vi "inject contour on intensity plot.vi"(5 "graph para":T1={"x offset"=-10.0, "y offset"=0.0, "x scale"=0.1, "y scale"=0.002}, 7 "Threshold":dbl, 11 "IV Intensity":dbl[][](array[numeric])=array201x1000[201000 elements]) -> (1 "Y":dbl[](array[numeric]), 2 "X":dbl[](array[numeric]), 3 "IV Intensity output":dbl[][](graph))   [LabVIEW 2024]
uses:
  graph para.ctl
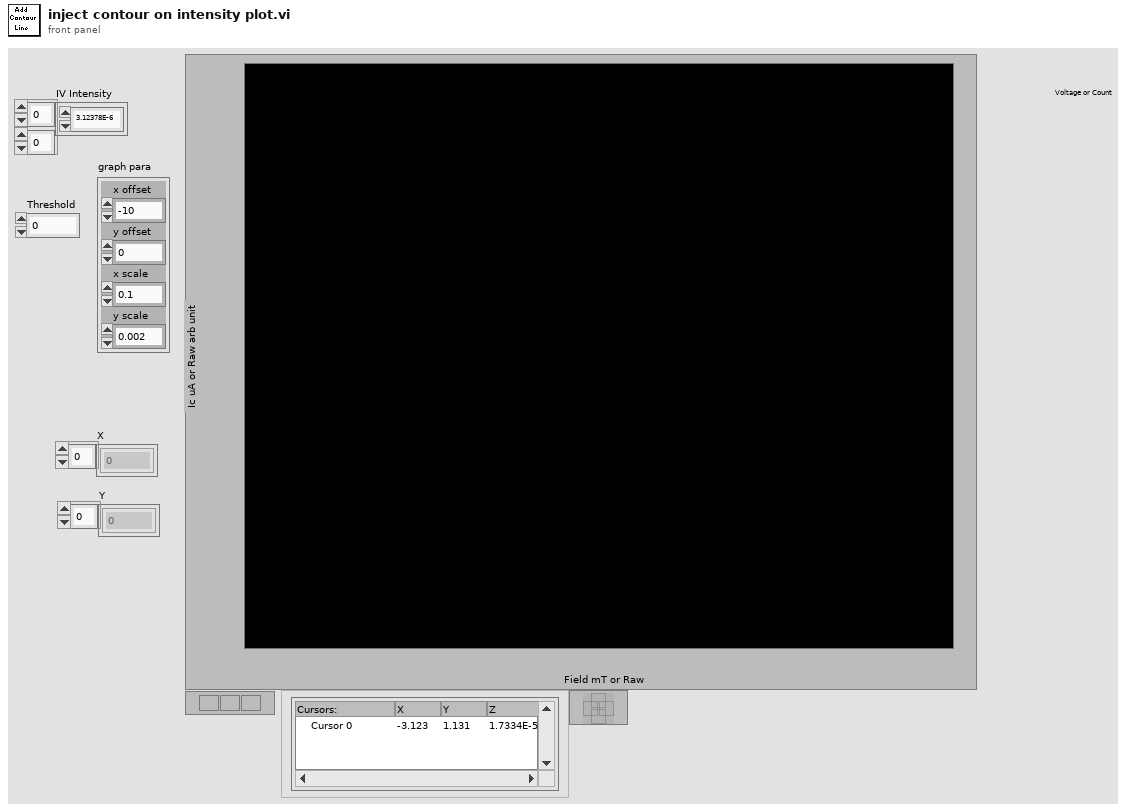
[diagram p1: front panel]
types:
  T1 = typedef "graph para.ctl" = cluster{"x offset":dbl, "y offset":dbl, "x scale":dbl, "y scale":dbl}
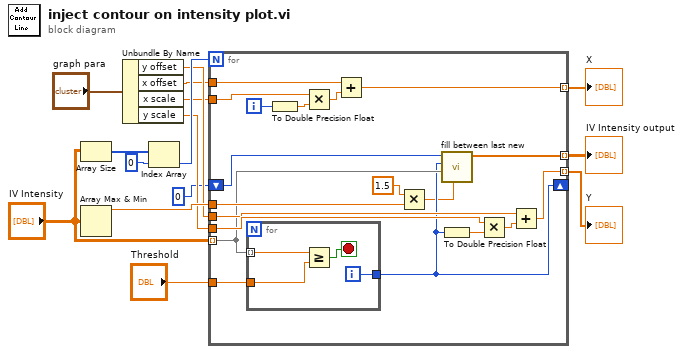
[diagram p0: block diagram]
diagram:
  n1 = Array Size(array="IV Intensity") -> (size(s)=w15:i32[])
  n2 = Array Max & Min(array="IV Intensity") -> (max value=w11:dbl)  [unwired: 3 out]
  n3 = Unbundle By Name("graph para") -> ("y offset"=w8:dbl, "x offset"=w7:dbl, "x scale"=w6:dbl, "y scale"=w5:dbl)
  n4 = Index Array(array=w15, index=0) -> (element=w13:i32)
  n5 = for {
    N: w13 -> [_]
    tunnel: w6 -> [w33]
    tunnel: w7 -> [w30]
    tunnel: w8 -> [w22]
    tunnel: w5 -> [w23]
    tunnel: "IV Intensity" -> [w20] mode=indexing
    tunnel: w11 -> [w29]
    tunnel: [w19] -> w10 mode=indexing
    tunnel: "Threshold" -> [w27]
    tunnel: [w26] -> w3 mode=indexing
    tunnel: [w21] -> w2 mode=indexing
    shift-right: [w17] -> _
    shift-left: 0 -> [w18]
    i -> [w34]
    n6 = for {
      tunnel: w20 -> [w38] mode=indexing
      tunnel: w27 -> [w37]
      tunnel: [w35] -> w17
      i -> [w35]
      stop <- w36 stop-if-true
      n7 = Greater Or Equal?(x=w38, y=w37) -> (x >= y?=w36:bool)
    }
    n8 = To Double Precision Float(number=w34) -> (double precision float=w32:dbl)
    n9 = Multiply(x=w33, y=w32) -> (x*y=w31:dbl)
    n10 = Add(x=w30, y=w31) -> (x+y=w26:dbl)
    n11 = Multiply(x=1.5, y=w29) -> (x*y=w16:dbl)
    n12 = call "fill between last new.vi"("value"=w16, "array in"=w20, "New"=w17, "Last"=w18) -> ("array out"=w19:dbl[])  [unwired: 7 in]
    n13 = To Double Precision Float(number=w17) -> (double precision float=w25:dbl)
    n14 = Multiply(x=w23, y=w25) -> (x*y=w24:dbl)
    n15 = Add(x=w22, y=w24) -> (x+y=w21:dbl)
  }
  "IV Intensity output" <- w10
  "X" <- w3
  "Y" <- w2
